vi "Login.vi"() -> ()   [LabVIEW 2020]
uses:
  System.Windows.Forms
  Global_Variable/Global.vi
  <userlib>/_MGI/Menu Building/MenuItemStatusChange/MGI_MenuItemStatusChange.lvclass
panel:
  in  "联机模式":enum16{"单机", "追溯"}(ring)
  in  "菜单":refnum<k24>(container)
  in  "登陆":bool
  in  "密   码":string
  in  "用户名":string
  out "数据库连接成功":bool
  # "NVH检测"
  # "数据库状态"
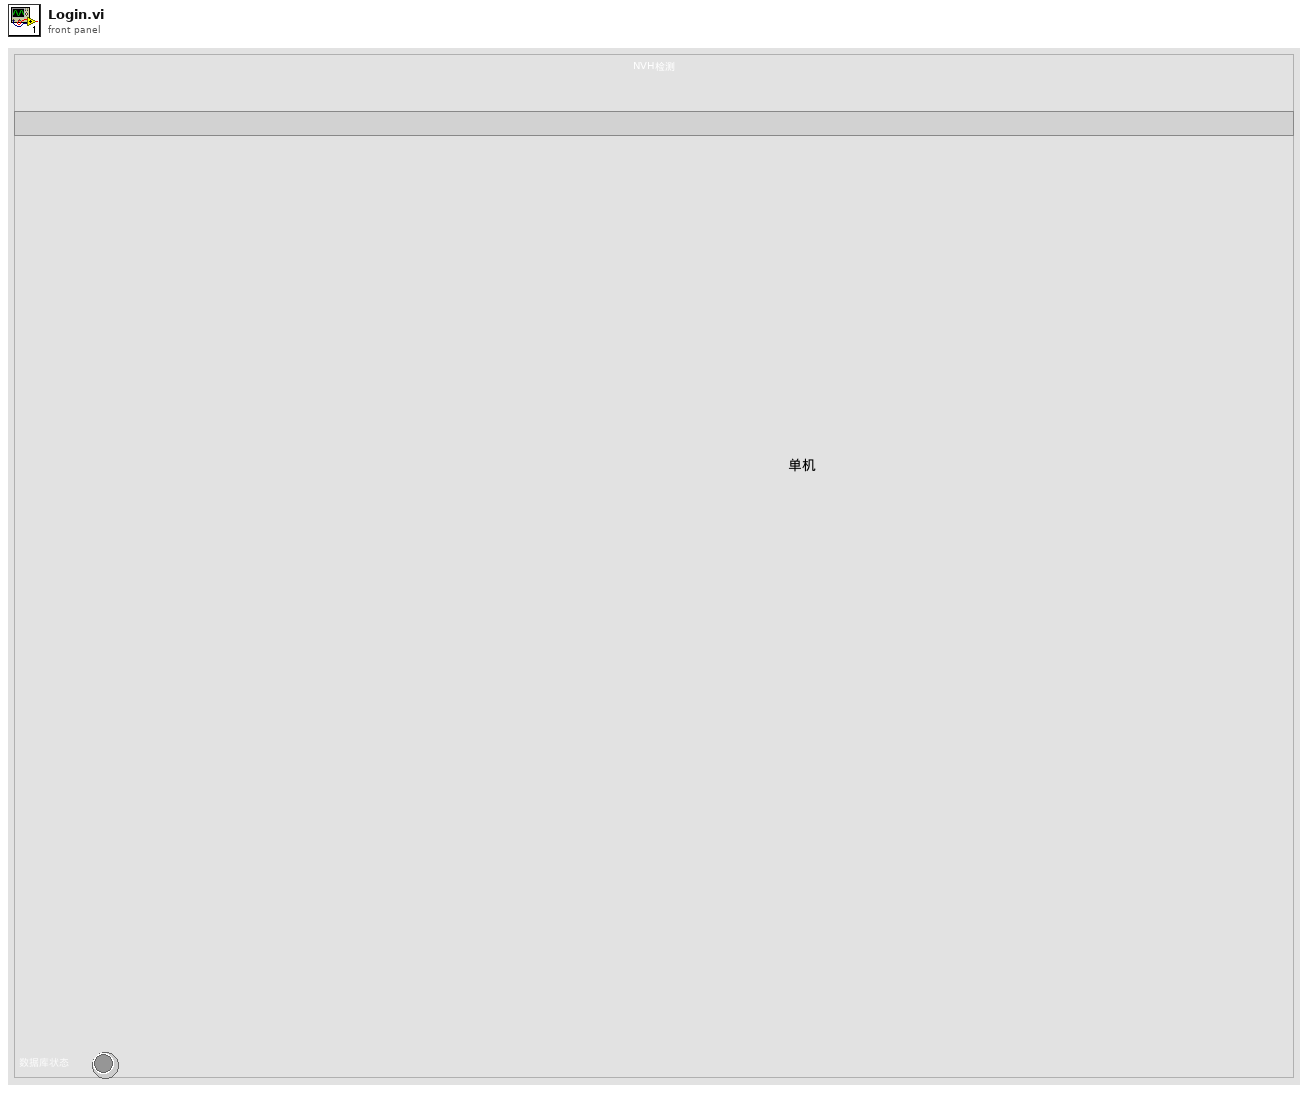
[diagram p1: front panel]
types:
  T1 = enum32{"Invalid", "Standard", "Closed", "Hidden", "Minimized", "Maximized"}
  T2 = cluster{"data[0]":string, "data[1]":string, "data[2]":string, "data[3]":string}
  T3 = typedef "eventvkey.ctl" = enum16{"ASCII", "Enter", "Return", "Shift", "Ctrl", "Alt", "Cmd", "Opt", "Caps", "NumLock", "Clear", "Break", "Up", "Down", "Left", "Right", "Insert", "Delete", "Home", "End", "PageUp", "PageDown", "Escape", "Help", "Pause", "ScrollLock", "F1", "F2", "F3", "F4", "F5", "F6", "F7", "F8", "F9", "F10", "F11", "F12", "F13", "F14", "F15", "F16", "F17", "F18", "F19", "F20", "F21", "F22", "F23", "F24", "Play", "VolumeUp", "VolumeDown", "Mute", "Two Byte Char"}
  T4 = cluster{"用户编号":string, "用户名":string, "用户密码(密文)":string, "用户权限":string}
  T5 = cluster{"操作员编号":string, "操作员姓名":string, "操作员权限":string, "联机模式":enum16{"单机", "追溯"}}
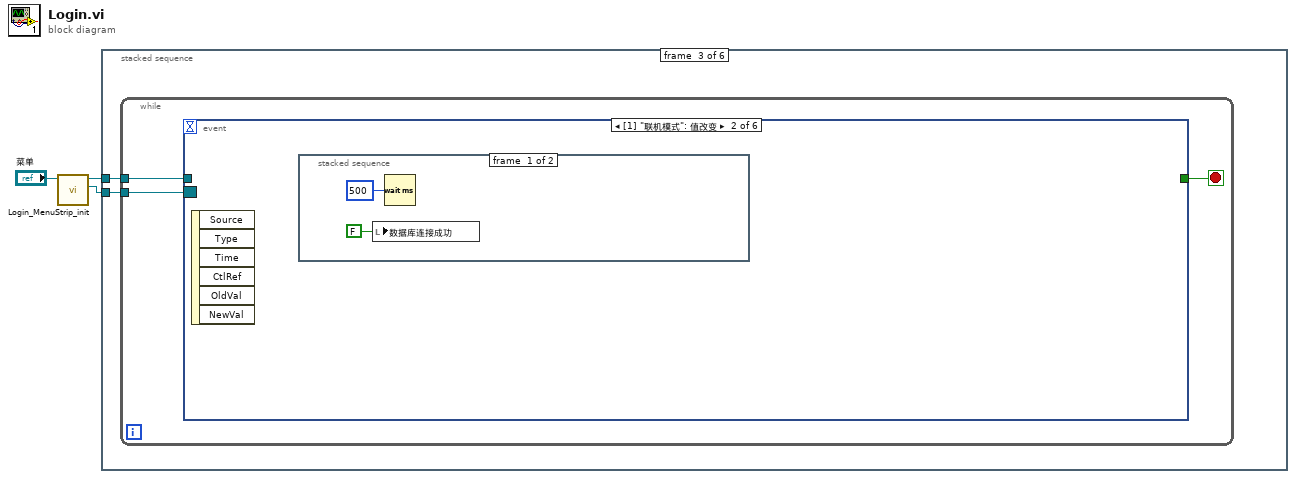
[diagram p0: block diagram]
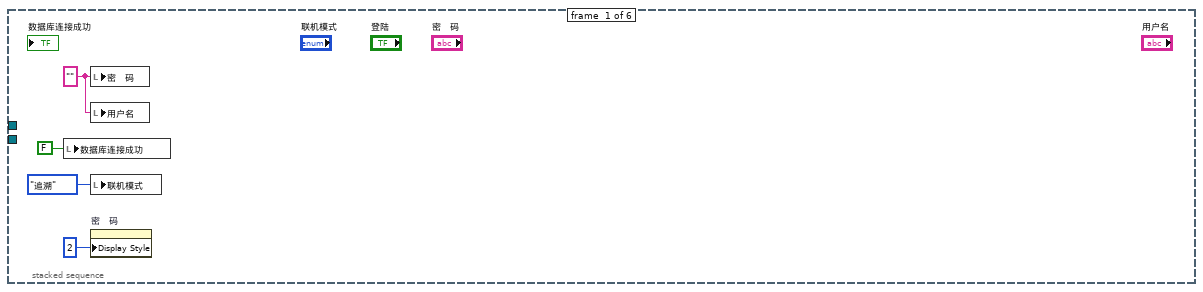
[diagram p2: hidden frame]
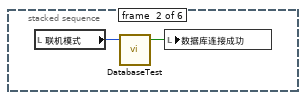
[diagram p3: hidden frame]
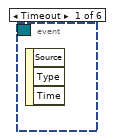
[diagram p4: hidden frame]
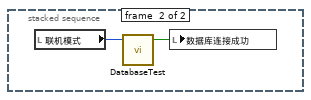
[diagram p5: hidden frame]
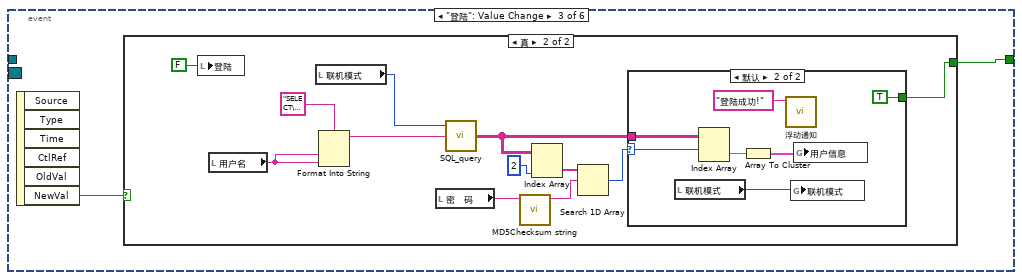
[diagram p6: hidden frame]
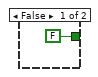
[diagram p7: hidden frame]
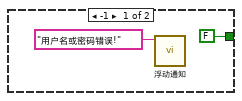
[diagram p8: hidden frame]
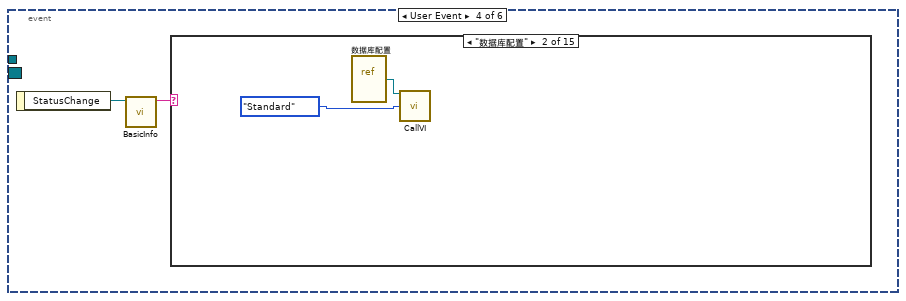
[diagram p9: hidden frame]
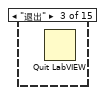
[diagram p11: hidden frame]
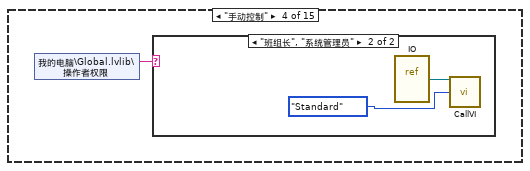
[diagram p12: hidden frame]
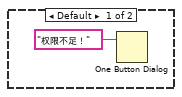
[diagram p13: hidden frame]
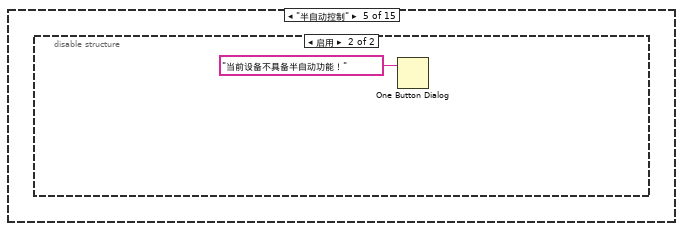
[diagram p14: hidden frame]
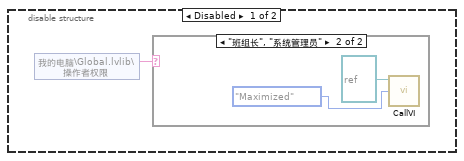
[diagram p15: hidden frame]
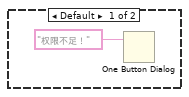
[diagram p16: hidden frame]
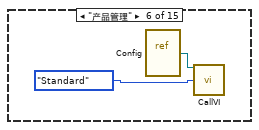
[diagram p17: hidden frame]
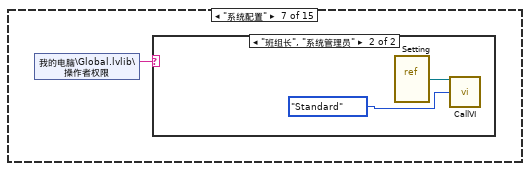
[diagram p18: hidden frame]
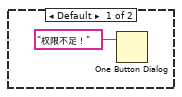
[diagram p19: hidden frame]
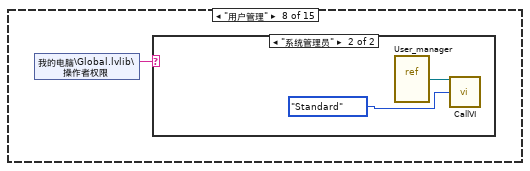
[diagram p20: hidden frame]
diagram:
  n1 = call "Login_MenuStrip_init.vi"("MenuStrip"="菜单") -> ("MenuStrip_Event"=w2:refnum<event-registration>, "Menu out"=w1:refnum<class "MGI_MenuStrip.lvclass">)  [unwired: 9 in]
  n2 = stacked-sequence {
    tunnel: w2 -> [_ _ w11 _ _ _]
    tunnel: w1 -> [_ _ w10 _ _ _]
    frame #0 {
      w6 = ""
      n3 = local write "数据库连接成功"(FALSE ("数据库连接成功")) -> ()
      n4 = local write "密   码"(w6) -> ()
      n5 = local write "用户名"(w6) -> ()
      n6 = local write "联机模式"(enum16{"单机", "追溯"}."追溯" ("联机模式")) -> ()
      n7 = property on="密   码" class="Str"("Display Style"=u32 2 ("显示样式")) -> ()  [unwired: 2 in, 2 out]
    }
    frame #1 {
      n8 = local read "联机模式"() -> (w8:enum16{"单机", "追溯"})
      n9 = call "DatabaseTest.vi"("联机模式"=w8) -> ("数据库连接成功"=w9:bool)  [unwired: 3 in, 1 out]
      n10 = local write "数据库连接成功"(w9) -> ()
    }
    frame #2 {
      n11 = while {
        tunnel: w11 -> [w13]
        tunnel: w10 -> [w12]
        stop <- w14 stop-if-true
        n12 = event shown="[1] \"联机模式\": 值改变" {
          selector: w13 -> [_ _ _ _ _ _]
          dyn-events: _ -> [_ _ _ _ _ _]
          timeout: _ -> [_ _ _ _ _ _]
          tunnel: [_ _ w19 _ _ TRUE] -> w14
          tunnel: w12 -> [_ _ _ _ _ _]
          event Timeout {
            n13 = event-data() -> ()  [unwired: 1 in, 3 out]
          }
          event "联机模式": Value Change {
            n14 = event-data() -> ()  [unwired: 1 in, 6 out]
            n15 = stacked-sequence {
              frame #0 {
                n16 = local write "数据库连接成功"(FALSE ("数据库连接成功")) -> ()
                n17 = Wait (ms)(milliseconds to wait=u32 500 ("等待时间（毫秒）")) -> ()  [unwired: 1 out]
              }
              frame #1 {
                n18 = local read "联机模式"() -> (w17:enum16{"单机", "追溯"})
                n19 = call "DatabaseTest.vi"("联机模式"=w17) -> ("数据库连接成功"=w18:bool)  [unwired: 3 in, 1 out]
                n20 = local write "数据库连接成功"(w18) -> ()
              }
            }
          }
          event "登陆": Value Change {
            n21 = event-data() -> ("NewVal"=w20:bool)  [unwired: 1 in, 5 out]
            n22 = case shown="真" w20 {
              tunnel: [FALSE w24] -> w19
              frame False {
              }
              frame True {
                n23 = local write "登陆"(FALSE ("确定")) -> ()
                n24 = local read "用户名"() -> (w30:string)
                n25 = local read "联机模式"() -> (w22:enum16{"单机", "追溯"})
                n26 = Format Into String(format string="SELECT\ndbo.[User].USER_EMPLOYEE_ID,\ndbo.[User].USER_NAME,\ndbo.[User].USER_PASSWD,\ndbo.[User].USER_PERMIT\n\nFROM\ndbo.[User]\nWHERE\ndbo.[User].USER_NAME = '%s' \nOR\ndbo.[User].USER_EMPLOYEE_ID = '%s'\n" ("格式字符串"), w30, w30) -> (resulting string=w27:string)  [unwired: 2 in, 1 out]
                n27 = local read "密   码"() -> (w31:string)
                n28 = call "SQL_query.vi"("SQL query"=w27, "联机模式"=w22) -> ("data"=w25:string[][])  [unwired: 2 in, 1 out]
                n29 = call <vilib>:"MD5Checksum string.vi"("Message String"=w31) -> ("MD5 message-digest"=w32:string)  [unwired: 10 in]
                n30 = Index Array(array=w25, index (col)=2 ("禁用的索引 (列)")) -> (element=w29:string[])  [unwired: 1 in]
                n31 = Search 1D Array(1D array=w29, element=w32) -> (index of element=w26:i32)  [unwired: 1 in]
                n32 = case shown="默认" w26 {
                  selector: w26 -> [_ w41]
                  tunnel: w25 -> [_ w42]
                  tunnel: [FALSE TRUE] -> w24
                  frame -1 {
                    n33 = call "浮动通知.vi"("通知内容"="用户名或密码错误!") -> ()  [unwired: 11 in]
                  }
                  frame Default {
                    n34 = local read "联机模式"() -> (w37:enum16{"单机", "追溯"})
                    n35 = Index Array(array=w42, index (row)=w41) -> (element=w39:string[])  [unwired: 1 in]
                    n36 = Array To Cluster(array=w39) -> (cluster=w36:T2)
                    n37 = call "浮动通知.vi"("通知内容"="登陆成功!") -> ()  [unwired: 11 in]
                    n38 = global write "Global.vi" "联机模式"(w37) -> ()
                    n39 = global write "Global.vi" "用户信息"(w36) -> ()
                  }
                }
              }
            }
          }
          event User Event {
            n40 = event-data() -> ("StatusChange"=w44:refnum<class "MGI_MenuItemStatusChange.lvclass">)  [unwired: 1 in]
            n41 = call <userlib>:"BasicInfo.vi"("MGI_MenuItemStatusChange in"=w44) -> ("Tag"=w43:string)  [unwired: 7 in, 3 out]
            n42 = case shown="\"数据库配置\"" w43 {
              frame "假", Default {
              }
              frame "数据库配置" {
                n43 = vi-ref "数据库配置.vi"() -> (w46:refnum<vi>)
                n44 = call "CallVI.vi"("VI引用"=w46, "状态"=T1."Standard") -> ()  [unwired: 12 in, 2 out]
              }
              frame "退出" {
                n45 = Quit LabVIEW() -> ()  [unwired: 1 in]
              }
              frame "手动控制" {
                n46 = shared-variable "我的电脑\\Global.lvlib\\操作者权限"() -> (w47:string)  [unwired: 1 in, 1 out]
                n47 = case shown="\"班组长\", \"系统管理员\"" w47 {
                  frame Default {
                    n48 = One Button Dialog(message="权限不足！" ("消息")) -> ()  [unwired: 1 in, 1 out]
                  }
                  frame "班组长", "系统管理员" {
                    n49 = vi-ref "IO.vi"() -> (w50:refnum<vi>)
                    n50 = call "CallVI.vi"("VI引用"=w50, "状态"=T1."Standard") -> ()  [unwired: 12 in, 2 out]
                  }
                }
              }
              frame "半自动控制" {
                n51 = disable-structure shown="启用" {
                  frame Disabled {
                    n52 = shared-variable "我的电脑\\Global.lvlib\\操作者权限"() -> (w51:string)  [unwired: 1 in, 1 out]
                    n53 = case shown="\"班组长\", \"系统管理员\"" w51 {
                      frame Default {
                        n54 = One Button Dialog(message="权限不足！" ("消息")) -> ()  [unwired: 1 in, 1 out]
                      }
                      frame "班组长", "系统管理员" {
                        n55 = call "CallVI.vi"("VI引用"=refnum<vi> refnum, "状态"=T1."Maximized") -> ()  [unwired: 12 in, 2 out]
                      }
                    }
                  }
                  frame Enabled {
                    n56 = One Button Dialog(message="当前设备不具备半自动功能！" ("消息")) -> ()  [unwired: 1 in, 1 out]
                  }
                }
              }
              frame "产品管理" {
                n57 = vi-ref "Config.vi"() -> (w57:refnum<vi>)
                n58 = call "CallVI.vi"("VI引用"=w57, "状态"=T1."Standard") -> ()  [unwired: 12 in, 2 out]
              }
              frame "系统配置" {
                n59 = shared-variable "我的电脑\\Global.lvlib\\操作者权限"() -> (w58:string)  [unwired: 1 in, 1 out]
                n60 = case shown="\"班组长\", \"系统管理员\"" w58 {
                  frame Default {
                    n61 = One Button Dialog(message="权限不足！" ("消息")) -> ()  [unwired: 1 in, 1 out]
                  }
                  frame "班组长", "系统管理员" {
                    n62 = vi-ref "Setting.vi"() -> (w61:refnum<vi>)
                    n63 = call "CallVI.vi"("VI引用"=w61, "状态"=T1."Standard") -> ()  [unwired: 12 in, 2 out]
                  }
                }
              }
              frame "用户管理" {
                n64 = shared-variable "我的电脑\\Global.lvlib\\操作者权限"() -> (w62:string)  [unwired: 1 in, 1 out]
                n65 = case shown="\"系统管理员\"" w62 {
                  frame Default {
                    n66 = One Button Dialog(message="权限不足！" ("消息")) -> ()  [unwired: 1 in, 1 out]
                  }
                  frame "系统管理员" {
                    n67 = vi-ref "User_manager.vi"() -> (w65:refnum<vi>)
                    n68 = call "CallVI.vi"("VI引用"=w65, "状态"=T1."Standard") -> ()  [unwired: 12 in, 2 out]
                  }
                }
              }
              frame "编码规则" {
                n69 = shared-variable "我的电脑\\Global.lvlib\\操作者权限"() -> (w66:string)  [unwired: 1 in, 1 out]
                n70 = case shown="\"班组长\", \"工艺管理员\", \"系统管理员\"" w66 {
                  frame Default {
                    n71 = One Button Dialog(message="权限不足！" ("消息")) -> ()  [unwired: 1 in, 1 out]
                  }
                  frame "班组长", "工艺管理员", "系统管理员" {
                    n72 = vi-ref "编码规则设置.vi"() -> (w69:refnum<vi>)
                    n73 = call "CallVI.vi"("VI引用"=w69, "状态"=T1."Standard") -> ()  [unwired: 12 in, 2 out]
                  }
                }
              }
              frame "易损件管理" {
                n74 = vi-ref "易损件管理.vi"() -> (w71:refnum<vi>)
                n75 = call "CallVI.vi"("VI引用"=w71, "状态"=T1."Standard") -> ()  [unwired: 12 in, 2 out]
              }
              frame "物料批次管理" {
                n76 = vi-ref "批次管理.vi"() -> (w73:refnum<vi>)
                n77 = call "CallVI.vi"("VI引用"=w73, "状态"=T1."Standard") -> ()  [unwired: 12 in, 2 out]
              }
              frame "报表" {
                n78 = call "文件对话框"("start path"=path "D:/report", "prompt"="打开报表", "pattern (all files)"="*.doc;*.docx", "pattern label"="Word 文档") -> ("selected path"=w74:path, "error out"=w75:errorcluster)  [unwired: 8 in, 2 out]
                n79 = case shown="无错误" w75 {
                  selector: w75 -> [w81 w83]
                  tunnel: w74 -> [w82 _]
                  frame No Error {
                    w80 = 1 items=["Normal", "Maximize", "Minimize"] ("cpubbs_WindowState")
                    n80 = call "Open_Word.vi"("File Path"=w82, "cpubbs_WindowState"=w80, "错误输入（无错误）"=w81) -> ()  [unwired: 12 in, 1 out]
                  }
                  frame Error {
                    n81 = call <vilib>:"Clear Errors.vi"("error in (no error)"=w83) -> ()  [unwired: 5 in, 2 out]
                  }
                }
              }
              frame "报警信息" {
                n82 = vi-ref "报警信息.vi"() -> (w85:refnum<vi>)
                n83 = call "CallVI.vi"("VI引用"=w85, "状态"=T1."Standard") -> ()  [unwired: 12 in, 2 out]
              }
              frame "关于" {
                n84 = vi-ref "About.vi"() -> (w87:refnum<vi>)
                n85 = call "CallVI.vi"("VI引用"=w87, "状态"=T1."Standard") -> ()  [unwired: 12 in, 2 out]
              }
              frame "操作演示" {
                n86 = call <vilib>:"Application Directory.vi"() -> ("Application Directory"=w90:path)
                n87 = Build Path(base path=w90, name or relative path="操作演示" ("名称或相对路径")) -> (appended path=w89:path)
                n88 = call "自动播放ppt.vi"("路径"=w89) -> ()  [unwired: 10 in, 1 out]
              }
            }
          }
          event Key Down {
            n89 = event-data() -> ("VKey"=w91:T3)  [unwired: 1 in, 9 out]
            n90 = case shown="\"Return\"" w91 {
              frame "ASCII", Default {
              }
              frame "Return" {
                n91 = property on="登陆" class="Bool (严格)"("Val(Sgnl)"=TRUE ("值(信号)")) -> ()  [unwired: 2 in, 2 out]
              }
            }
          }
          event Panel Close {
            n92 = event-data() -> ()  [unwired: 1 in, 4 out]
            n93 = Quit LabVIEW() -> ()  [unwired: 1 in]
          }
        }
      }
    }
    frame #3 {
      n94 = global read "Global.vi" "用户信息"() -> (w98:T4)
      n95 = global read "用户信息.vi" "用户信息"() -> (w97:T5)
      n96 = Unbundle By Name(w98) -> ("用户编号"=w99:string, "用户权限"=w95:string)
      n97 = call "Get_Device_ID.vi"() -> ("Device_ID"=w94:string)  [unwired: 10 in, 1 out]
      n98 = Bundle By Name(cluster=w97, "操作员权限"=w95) -> (w96:T5)
      n99 = call "Get_USER_ID.vi"("USER_EMPLOYEE_ID"=w99) -> ("USER_ID"=w100:string)  [unwired: 9 in, 1 out]
      n100 = global write "用户信息.vi" "用户信息"(w96) -> ()
      n101 = global write "追溯Global.vi" "USER_ID"(w100) -> ()
      n102 = global write "追溯Global.vi" "DEVICE_ID"(w94) -> ()
    }
    frame #4 {
      n103 = vi-ref "Main.vi"() -> (w102:refnum<vi>)
      n104 = call "CallVI.vi"("VI引用"=w102, "状态"=T1."Maximized") -> ()  [unwired: 12 in, 2 out]
    }
    frame #5 {
      n105 = control-ref of="本VI"() -> (w103:refnum<vi>)
      n106 = invoke class="VI" method="FP.Close"(reference=w103) -> (reference out=w104:refnum<vi>, error out=w105:errorcluster)  [unwired: 2 in, 1 out]
      n107 = Close Reference(reference=w104, error in (no error)=w105) -> ()  [unwired: 1 out]
    }
  }
